vi "Controle_Manip_Main_GUI_Backup2.vi"() -> ()   [LabVIEW 2019] (continued)
                                }
                                frame #2 {
                                n2013 = local read "BackgroundSpec"() -> (w2482:dbl[])
                                n2014 = call-poly <vilib>:"Mean.vi"("X"=w2482) -> ("mean"=w2484:dbl)  [unwired: 1 out]
                                n2015 = Negate(x=w2484) -> (-x=w2483:dbl)
                                n2016 = property on="CCD 1D Spectrum Main" class="XYGraph (strict)"("YScale.Offset"=w2483) -> ()  [unwired: 2 in, 2 out]
                                }
                                frame #3 {
                                n2017 = local write "Background taken?"(TRUE ("Background taken?")) -> ()
                                n2018 = property on="Background substract" class="Enum (strict)"("Value"=enum16{"None", "Shutter"}."None" ("Background substract")) -> ()  [unwired: 2 in, 2 out]
                                }
                                }
                                }
                                frame "Image" {
                                n2019 = stacked-sequence {
                                tunnel: w2488 -> [_ w2496]
                                tunnel: w2487 -> [_ w2494]
                                frame #0 {
                                n2020 = property on="CCD 1D Spectrum Main" class="XYGraph (strict)"("Visible"=FALSE) -> ()  [unwired: 2 in, 2 out]
                                n2021 = property on="CCD 2D Image Main" class="IntGraph (strict)"("Visible"=TRUE) -> ()  [unwired: 2 in, 2 out]
                                }
                                frame #1 {
                                n2022 = local read "Wavelength calibration"() -> (w2495:dbl[])
                                n2023 = local read "CCD ROI"() -> (w2491:T20)
                                n2024 = call "PrepareData4Graph.vi"("Wavelength nm"=w2495, "DataLF"=w2496, "CCD ROI"=w2491, "AcqMode"=w2494, "Data type"=T30."Spectre") -> ("Intensity Graph"=w2493:dbl[][])  [unwired: 2 in, 3 out]
                                n2025 = local write "CCD 2D Image Main"(w2493) -> ()
                                }
                                }
                                }
                                }
                              }
                              frame True {
                              }
                            }
                          }
                          frame #1 {
                            w2521 = 1 ("Active X Scale")
                            w2522 = 0
                            # "prep axes for graphs (a nightmare in LabVIEW to not display 1...N but rather Volts or um)"
                            n2026 = local read "Scan X Res. (V)"() -> (w2526:dbl)
                            n2027 = local read "Scan X Tot. Length (V)"() -> (w2524:dbl)
                            n2028 = local read "Scan X Res. (V)"() -> (w2555:dbl)
                            n2029 = local read "Scan X Center (V)"() -> (w2523:dbl)
                            n2030 = local read "Scan X Center (V)"() -> (w2557:dbl)
                            n2031 = local read "Scan Y Center (V)"() -> (w2549:dbl)
                            n2032 = local read "Scan Y Res. (V)"() -> (w2548:dbl)
                            n2033 = local read "Scan Y Tot. Length"() -> (w2551:dbl)
                            n2034 = local read "Scan X Tot. Length (V)"() -> (w2556:dbl)
                            n2035 = local read "V2um"() -> (w2525:dbl)
                            n2036 = call "V2um.vi"("Numeric"=w2526, "V2um"=w2525) -> ("x*y"=w2530:dbl)
                            n2037 = call "V2um.vi"("Numeric"=w2524, "V2um"=w2525) -> ("x*y"=w2527:dbl)
                            n2038 = call "V2um.vi"("Numeric"=w2523, "V2um"=w2525) -> ("x*y"=w2531:dbl)
                            n2039 = Divide(x=w2527, y=w2530) -> (x/y=w2528:dbl)
                            n2040 = local read "Scan Y Res. (V)"() -> (w2537:dbl)
                            n2041 = Divide(x=w2551, y=w2548) -> (x/y=w2552:dbl)
                            n2042 = Increment(x=w2552) -> (x+1=w2550:dbl)
                            n2043 = Increment(x=w2528) -> (x+1=w2529:dbl)
                            n2044 = call "AxXYGraph.vi"("dx"=w2530, "N"=w2529, "x0"=w2531) -> ("Multiplier"=w2520:dbl, "Offset"=w2519:dbl)
                            n2045 = local read "Scan Y Tot. Length"() -> (w2539:dbl)
                            n2046 = Divide(x=w2556, y=w2555) -> (x/y=w2554:dbl)
                            n2047 = local read "Scan Y Center (V)"() -> (w2540:dbl)
                            n2048 = call "AxXYGraph.vi"("dx"=w2548, "N"=w2550, "x0"=w2549) -> ("Multiplier"=w2547:dbl, "Offset"=w2546:dbl)
                            n2049 = Increment(x=w2554) -> (x+1=w2553:dbl)
                            n2050 = call "AxXYGraph.vi"("dx"=w2555, "N"=w2553, "x0"=w2557) -> ("Multiplier"=w2544:dbl, "Offset"=w2545:dbl)
                            n2051 = local read "BackgroundSpec"() -> (w2543:dbl[])
                            n2052 = local read "V2um"() -> (w2538:dbl)
                            n2053 = call "V2um.vi"("Numeric"=w2537, "V2um"=w2538) -> ("x*y"=w2533:dbl)
                            n2054 = call "V2um.vi"("Numeric"=w2539, "V2um"=w2538) -> ("x*y"=w2536:dbl)
                            n2055 = call "V2um.vi"("Numeric"=w2540, "V2um"=w2538) -> ("x*y"=w2532:dbl)
                            n2056 = Divide(x=w2536, y=w2533) -> (x/y=w2535:dbl)
                            n2057 = Increment(x=w2535) -> (x+1=w2534:dbl)
                            n2058 = call "AxXYGraph.vi"("dx"=w2533, "N"=w2534, "x0"=w2532) -> ("Multiplier"=w2518:dbl, "Offset"=w2517:dbl)
                            n2059 = call-poly <vilib>:"Mean.vi"("X"=w2543) -> ("mean"=w2542:dbl)  [unwired: 1 out]
                            n2060 = property on="XY Intensity Map" class="IntGraph (strict)"("ActXScl"=w2522, "XScale.Multiplier"=w2544, "XScale.Offset"=w2545, "ActYScl"=w2522, "YScale.Multiplier"=w2547, "YScale.Offset"=w2546) -> ()  [unwired: 2 in, 2 out]
                            n2061 = property on="XY Intensity Map" class="IntGraph (strict)"("ActXScl"=w2521, "XScale.Multiplier"=w2520, "XScale.Offset"=w2519, "ActYScl"=w2521, "YScale.Multiplier"=w2518, "YScale.Offset"=w2517) -> ()  [unwired: 2 in, 2 out]
                            n2062 = Negate(x=w2542) -> (-x=w2541:dbl)
                            n2063 = property on="CCD 1D Spectrum XY Map" class="XYGraph (strict)"("YScale.Offset"=w2541) -> ()  [unwired: 2 in, 2 out]
                          }
                          frame #2 {
                            w2577 = 1 ("Active Y Scale")
                            w2587 = FALSE
                            w2588 = TRUE ("Visible")
                            # "nightmare part II"
                            n2064 = local read "Scan X Res. (V)"() -> (w2565:dbl)
                            n2065 = local read "Scan Y Center (V)"() -> (w2582:dbl)
                            n2066 = local read "Scan X Center (V)"() -> (w2583:dbl)
                            n2067 = local read "Scanning Mode"() -> (w2592:T21)
                            n2068 = local read "Scan Y Res. (V)"() -> (w2566:dbl)
                            n2069 = local read "Scan Fast Axis"() -> (w2593:enum16{"Y", "X"})
                            n2070 = local read "Scan XY Map Params"() -> (w2595:refnum<vi>[])
                            n2071 = property on="Save XY Map" class="Bool (strict)"("Visible"=w2587) -> ()  [unwired: 2 in, 2 out]
                            n2072 = property on="Acquire XY Map" class="Bool (strict)"("Visible"=w2587) -> ()  [unwired: 2 in, 2 out]
                            n2073 = local read "Scan X Tot. Length (V)"() -> (w2580:dbl)
                            n2074 = control-ref of="MasterPause"() -> (w2562:refnum<vi>)
                            n2075 = local read "Scan Y Tot. Length"() -> (w2581:dbl)
                            n2076 = property on="CCD 1D Spectrum Main Energy Scale" class="XYGraph (strict)"() -> ("XScale.MarkerVals[]"=w2586:dbl[], "XScale.Maximum"=w2585:dbl, "XScale.Minimum"=w2584:dbl)  [unwired: 2 in, 2 out]
                            n2077 = property on="Experiment Graph Controls" class="TabCtl (strict)"("Value"=T25."XY Intensity Map" ("Experiment Graph Controls")) -> ()  [unwired: 2 in, 2 out]
                            n2078 = property class="Bool (strict)"(reference=w2562, "Visible"=TRUE) -> ()  [unwired: 1 in, 2 out]
                            n2079 = call "Enable&Disable_Controls.vi"("Enum"=enum16{"Enabled", "Disabled", "Disabled&Grayed"}."Disabled&Grayed", "References"=w2595) -> ()  [unwired: 1 in]
                            n2080 = Bundle("Scan Fast Axis"=w2593, "Scanning Mode"=w2592, "Scan X Center (V)"=w2583, "Scan X Res. (V)"=w2565, "Scan X Tot. Length (V)"=w2580, "Scan Y Center (V)"=w2582, "Scan Y Res. (V)"=w2566, "Scan Y Tot. Length"=w2581) -> (→"Params XY Map SubVI":T23)  [unwired: 1 in]
                            n2081 = property on="Scan Main Progess Bar" class="Slide (strict)"("Visible"=TRUE, "Value"=u8 0 ("Scan XY Map Progess Bar")) -> ()  [unwired: 2 in, 2 out]
                            n2082 = control-ref of="MasterStop"() -> (w2559:refnum<vi>)
                            n2083 = local read "V2um"() -> (w2564:dbl)
                            n2084 = property on="CCD 1D XY Map Spectrum Main Energy Scale" class="XYGraph (strict)"("XScale.MarkerVals[]"=w2586, "XScale.Maximum"=w2585, "XScale.Minimum"=w2584, "XScale.UniformMarker"=TRUE ("X Scale.Uniform Marker Spacing?")) -> ()  [unwired: 2 in, 2 out]
                            n2085 = property class="Bool (strict)"(reference=w2559, "Visible"=TRUE) -> ()  [unwired: 1 in, 2 out]
                            n2086 = call "AxxXY.vi"("Y Tot"=w2581, "X Tot"=w2580, "Y Res"=w2566, "Y Center"=w2582, "X Res"=w2566, "X Center"=w2583) -> ("YMIN"=w2568:dbl, "YMAX"=w2567:dbl, "XMIN"=w2569:dbl, "XMAX"=w2570:dbl)
                            n2087 = call "V2um.vi"("Numeric"=w2569, "V2um"=w2564) -> ("x*y"=w2575:dbl)
                            n2088 = call "V2um.vi"("Numeric"=w2570, "V2um"=w2564) -> ("x*y"=w2576:dbl)
                            n2089 = call "V2um.vi"("Numeric"=w2568, "V2um"=w2564) -> ("x*y"=w2574:dbl)
                            n2090 = call "V2um.vi"("Numeric"=w2567, "V2um"=w2564) -> ("x*y"=w2573:dbl)
                            n2091 = call "V2um.vi"("Numeric"=w2566, "V2um"=w2564) -> ("x*y"=w2572:dbl)
                            n2092 = call "V2um.vi"("Numeric"=w2565, "V2um"=w2564) -> ("x*y"=w2571:dbl)
                            n2093 = property on="Elapsed (s)" class="DigNum (strict)"("Visible"=w2588) -> ()  [unwired: 2 in, 2 out]
                            n2094 = property on="Expected (s)" class="DigNum (strict)"("Visible"=w2588) -> ()  [unwired: 2 in, 2 out]
                            n2095 = property on="XY Intensity Map" class="IntGraph (strict)"("ActYScl"=0 ("Active Y Scale"), "ActXScl"=0 ("Active X Scale"), "XScale.Maximum"=w2570, "XScale.Minimum"=w2569, "YScale.Minimum"=w2568, "YScale.Maximum"=w2567, "YScale.Increment"=w2566, "XScale.Increment"=w2565) -> ()  [unwired: 2 in, 2 out]
                            n2096 = property on="XY Intensity Map" class="IntGraph (strict)"("ActYScl"=w2577, "ActXScl"=w2577, "XScale.Maximum"=w2576, "XScale.Minimum"=w2575, "YScale.Minimum"=w2574, "YScale.Maximum"=w2573, "YScale.Increment"=w2572, "XScale.Increment"=w2571) -> ()  [unwired: 2 in, 2 out]
                          }
                          frame #3 {
                            w2596 = 0 ("Active X Scale")
                            n2097 = property on="XY Intensity Map" class="IntGraph (strict)"("ActXScl"=w2596, "ActYScl"=w2596) -> ()  [unwired: 2 in, 2 out]
                          }
                          frame #4 {
                            n2098 = local read "Excitation Wavelength (nm)"() -> (w2606:dbl)
                            n2099 = local read "FSM Y Task"() -> (w2617:refnum<k21>)
                            n2100 = local read "FSM X Task"() -> (w2618:refnum<k21>)
                            n2101 = local read "Photodiode handle out"() -> (w2607:refnum<visa-resource-name>)
                            n2102 = local read "LightField Automation out"() -> (w2609:refnum<class "LightField Automation.lvclass">)
                            n2103 = local read "Photodiode error out"() -> (w2605:errorcluster)
                            n2104 = local read "Excitation Wavelength (nm)"() -> (w2613:dbl)
                            n2105 = local read "LightField Automation error out"() -> (w2608:errorcluster)
                            n2106 = local read "KCube Shutter On?"() -> (w2610:bool)
                            n2107 = local read "BackgroundSpec"() -> (w2599:dbl[])
                            n2108 = local read "Accumulations"() -> (w2614:dbl)
                            n2109 = local read "Acq Time (ms)"() -> (w2615:dbl)
                            n2110 = local read "Acq Mode"() -> (w2612:T3)
                            n2111 = local read "CCD ROI"() -> (w2611:T20)
                            n2112 = Bundle("LightField Automation out"=w2609, "LightField Automation error out"=w2608, "FSM X Task"=w2618, "FSM Y Task"=w2617) -> (→"Scan XY Map Handles":T12)  [unwired: 1 in]
                            n2113 = call <instrlib>:"TLPM Set Wavelength.vi"("error in (no error)"=w2605, "Wavelength (0.0)"=w2606, "instrument handle"=w2607) -> ("error out"=w2604:errorcluster, "instrument handle out"=w2603:refnum<visa-resource-name>)  [unwired: 7 in]
                            n2114 = call <instrlib>:"TLPM Measure Power.vi"("error in (no error)"=w2604, "instrument handle"=w2603) -> ("error out"=w2601:errorcluster, "Power"=w2600:dbl, "instrument handle out"=w2602:refnum<visa-resource-name>)  [unwired: 7 in]
                            n2115 = local write "Photodiode handle out"(w2602) -> ()
                            n2116 = local write "Photodiode error out"(w2601) -> ()
                            n2117 = local write "Excitation Power (uW)"(w2600) -> ()
                            n2118 = control-ref of="Display Mode"() -> (w2598:refnum<vi>)
                            n2119 = Bundle("Acq Time (ms)"=w2615, "Accumulations"=w2614, "Excitation Wavelength (nm)"=w2613, "Acq Mode"=w2612, "CCD ROI"=w2611, "KCube Shutter On?"=w2610, "Power"=w2600, "BackgroundSpec"=w2599, "Display Mode"=w2598) -> (→"Scan XY Map Exp Params SubVI":T7)  [unwired: 1 in]
                            n2120 = case shown="True" w2610 {
                              selector: w2610 -> [_ w2619]
                              frame False {
                              }
                              frame True {
                                n2121 = control-ref of="Shutter Ctrls"() -> (w2622:refnum<vi>)
                                n2122 = property class="Ring (strict)"(reference=w2622) -> ("Value"=w2623:u16)  [unwired: 1 in, 2 out]
                                n2123 = control-ref of="KCube Shutter Device Reference"() -> (w2621:refnum<vi>)
                                n2124 = Equal?(x=w2623, y=u16 0) -> (x = y?=w2624:bool)
                                n2125 = case shown="True" w2624 {
                                tunnel: w2621 -> [_ w2627]
                                tunnel: w2622 -> [_ w2626]
                                tunnel: w2619 -> [_ w2625]
                                frame False {
                                }
                                frame True {
                                n2126 = call "Shutter.vi"("KCube Shutter Device Reference 2"=w2627, "Shutter Ctrls 2"=w2626, "Shutter on?"=w2625) -> ()
                                }
                                }
                              }
                            }
                          }
                          frame #5 {
                            n2127 = local read "Scan XY Map Exp Params SubVI"() -> (w2630:T7)
                            n2128 = local read "Scan XY Map References"() -> (w2631:T9)
                            n2129 = local read "Params XY Map SubVI"() -> (w2635:T23)
                            n2130 = local read "Scan XY Map Handles"() -> (w2634:T12)
                            n2131 = call "ScanFSM_v2.vi"("Scan XY Map References"=w2631, "Scan XY Map Handles"=w2634, "Params XY Map SubVI"=w2635, "Scan XY Map Exp Params SubVI"=w2630) -> ("Handles Out"=w2632:T36, "Data"=w2633:i32[][], "XYPos Indices"=w2629:i32[][], "XYPositions"=→"XYPositions":dbl[][])  [unwired: 12 in]
                            n2132 = local write "Scan XY Map Handles"(w2632) -> ()
                            n2133 = local write "XYMap Data"(w2633) -> ()
                            n2134 = local write "XYPos Indices"(w2629) -> ()
                          }
                          frame #6 {
                            n2135 = local read "Scan XY Map Handles"() -> (w2641:T12)
                            n2136 = local read "Scan Y Center (V)"() -> (w2636:dbl)
                            n2137 = local read "Scan X Center (V)"() -> (w2638:dbl)
                            n2138 = local read "KCube Shutter On?"() -> (w2643:bool)
                            n2139 = control-ref of="Shutter Ctrls"() -> (w2645:refnum<vi>)
                            n2140 = local read "FSM X Task"() -> (w2642:refnum<k21>)
                            n2141 = local read "FSM Y Task"() -> (w2637:refnum<k21>)
                            n2142 = control-ref of="KCube Shutter Device Reference"() -> (w2644:refnum<vi>)
                            n2143 = call "Shutter.vi"("KCube Shutter Device Reference 2"=w2644, "Shutter Ctrls 2"=w2645, "Shutter on?"=w2643) -> ()
                            n2144 = call "FSMGoTo.vi"("Target Value (V)"=w2638, "FSM Task"=w2642) -> ()  [unwired: 1 out]
                            n2145 = call "FSMGoTo.vi"("Target Value (V)"=w2636, "FSM Task"=w2637) -> ()  [unwired: 1 out]
                            n2146 = local write "Scan X Readout (V)"(w2638) -> ()
                            n2147 = Unbundle By Name(w2641) -> ("LightField Automation out"=w2640:refnum<class "LightField Automation.lvclass">, "LightField Automation error out"=w2639:errorcluster)
                            n2148 = property on="XY Intensity Map" class="IntGraph (strict)"("Cursor.Cursor X"=w2638) -> ()  [unwired: 2 in, 2 out]
                            n2149 = local write "Scan Y Readout (V)"(w2636) -> ()
                            n2150 = property on="XY Intensity Map" class="IntGraph (strict)"("Cursor.Cursor Y"=w2636) -> ()  [unwired: 2 in, 2 out]
                            n2151 = local write "LightField Automation error out"(w2639) -> ()
                            n2152 = local write "LightField Automation out"(w2640) -> ()
                          }
                          frame #7 {
                            w2646 = T28."Disabled and Grayed Out" ("Disabled")
                            w2659 = FALSE ("Visible")
                            n2153 = local read "Scan XY Map Params"() -> (w2663:refnum<vi>[])
                            n2154 = local read "Auto< ?"() -> (w2652:bool)
                            n2155 = local write "Acquire XY Map"(FALSE ("Acquire XY Map")) -> ()
                            n2156 = local write "Save XY Map"(FALSE ("Acquire XY Map")) -> ()
                            n2157 = case shown="True" w2652 {
                              tunnel: [TRUE FALSE] -> w2651
                              frame False {
                              }
                              frame True {
                              }
                            }
                            n2158 = call "Enable&Disable_Controls.vi"("Enum"=enum16{"Enabled", "Disabled", "Disabled&Grayed"}."Enabled", "References"=w2663) -> ()  [unwired: 1 in]
                            n2159 = property on="Acquire XY Map" class="Bool (strict)"("Visible"=TRUE, "Value"=FALSE ("Acquire XY Map")) -> ()  [unwired: 2 in, 2 out]
                            n2160 = local write "ExportMapPosition?"(TRUE ("ExportMapPosition?")) -> ()
                            n2161 = disable-structure shown="Disabled" {
                              disable-tunnel: w2659 -> [w2666 _]
                              frame Disabled {
                                n2162 = property on="Scan Main Progess Bar" class="Slide (strict)"("Visible"=w2666) -> ()  [unwired: 2 in, 2 out]
                              }
                              frame Enabled {
                              }
                            }
                            n2163 = property on="Save XY Map" class="Bool (strict)"("Visible"=w2651) -> ()  [unwired: 2 in, 2 out]
                            n2164 = property on="Elapsed (s)" class="DigNum (strict)"("Visible"=w2659) -> ("Value"=w2649:dbl)  [unwired: 2 in, 2 out]
                            n2165 = control-ref of="MasterStop"() -> (w2654:refnum<vi>)
                            n2166 = control-ref of="Scanning Mode"() -> (w2648:refnum<vi>)
                            n2167 = control-ref of="Scan Fast Axis"() -> (w2647:refnum<vi>)
                            n2168 = control-ref of="MasterPause"() -> (w2655:refnum<vi>)
                            n2169 = local write "Scan Main Progess Bar"(u8 0 ("Scan Main Progess Bar")) -> ()
                            n2170 = control-ref of="ExperimentStopped?"() -> (w2653:refnum<vi>)
                            n2171 = call "CheckStopAndReset.vi"("ExperimentStopped?"=w2653, "MasterStop"=w2654, "MasterPause"=w2655) -> ()
                            n2172 = property on="Expected (s)" class="DigNum (strict)"("Value"=w2649) -> ()  [unwired: 2 in, 2 out]
                            n2173 = property class="Enum (strict)"(reference=w2647, "DisabledEnum"=w2646) -> ()  [unwired: 1 in, 2 out]
                            n2174 = property class="Enum (strict)"(reference=w2648, "DisabledEnum"=w2646) -> ()  [unwired: 1 in, 2 out]
                          }
                        }
                      }
                      frame "Acquire Contrast test array of references" {
                        n2175 = stacked-sequence {
                          frame #0 {
                            w2669 = FALSE
                            w2670 = TRUE
                            w2678 = FALSE ("Acq Cont")
                            w2675 = FALSE ("Acq Cont")
                            n2176 = property on="CCD 1D Spectrum Main" class="XYGraph (strict)"() -> ("XScale.Maximum"=w2674:dbl, "XScale.Minimum"=w2673:dbl, "YScale.Minimum"=w2672:dbl, "YScale.Maximum"=w2671:dbl)  [unwired: 2 in, 2 out]
                            n2177 = property on="Acquire Contrast" class="Bool (strict)"("Visible"=w2669) -> ()  [unwired: 2 in, 2 out]
                            n2178 = property on="Save Contrast" class="Bool (strict)"("Visible"=w2669) -> ()  [unwired: 2 in, 2 out]
                            n2179 = property on="Scan Linear Stage Progess Bar" class="Slide (strict)"("Visible"=TRUE, "Value"=u8 0 ("Scan Linear Stage Progess Bar")) -> ()  [unwired: 2 in, 2 out]
                            n2180 = property on="Pause Contrast" class="Bool (strict)"("Visible"=w2670) -> ()  [unwired: 2 in, 2 out]
                            n2181 = property on="Stop Contrast" class="Bool (strict)"("Visible"=w2670) -> ()  [unwired: 2 in, 2 out]
                            n2182 = property on="Contrast 1D Spectrum" class="XYGraph (strict)"("XScale.Maximum"=w2674, "XScale.Minimum"=w2673, "YScale.Minimum"=w2672, "YScale.Maximum"=w2671) -> ()  [unwired: 2 in, 2 out]
                            n2183 = local read "Scan Contrast Ctrls"() -> (w2679:refnum<vi>[])
                            n2184 = property on="Experiment Graph Controls" class="TabCtl (strict)"("Value"=T25."Contrast" ("Experiment Graph Controls")) -> ()  [unwired: 2 in, 2 out]
                            n2185 = property on="Scan Linear Stage Progess Bar" class="Slide (strict)"("Visible"=TRUE) -> ()  [unwired: 2 in, 2 out]
                            n2186 = call "Enable&Disable_Controls.vi"("Enum"=enum16{"Enabled", "Disabled", "Disabled&Grayed"}."Disabled&Grayed", "References"=w2679) -> ()  [unwired: 1 in]
                            n2187 = local write "Acquire Contrast"(w2675) -> ()
                            n2188 = local write "Save Contrast"(w2675) -> ()
                            n2189 = local write "Pause Contrast"(w2678) -> ()
                            n2190 = local write "Stop Contrast"(w2678) -> ()
                          }
                          frame #1 {
                            n2191 = local read "ESP 301 COM Port"() -> (w2694:refnum<visa-resource-name>)
                            n2192 = local read "Photodiode handle out"() -> (w2692:refnum<visa-resource-name>)
                            n2193 = local read "Photodiode error out"() -> (w2691:errorcluster)
                            n2194 = local read "LightField Automation error out"() -> (w2681:errorcluster)
                            n2195 = local read "LinTFine End Pos (usteps)"() -> (w2698:dbl)
                            n2196 = local read "LinTFines Step Pos (usteps)"() -> (w2699:dbl)
                            n2197 = local read "LinTFine Start Pos (usteps)"() -> (w2700:dbl)
                            n2198 = local read "PZC200 Instrument Channel"() -> (w2696:string)
                            n2199 = local read "LinT End pos (mm)"() -> (w2701:dbl)
                            n2200 = local read "LightField Automation out"() -> (w2682:refnum<class "LightField Automation.lvclass">)
                            n2201 = local read "LinT Step Pos (mm)"() -> (w2702:dbl)
                            n2202 = local read "LinT Start Pos (mm)"() -> (w2703:dbl)
                            n2203 = local read "ESP 301 Error"() -> (w2693:errorcluster)
                            n2204 = local read "PZC Error"() -> (w2695:errorcluster)
                            n2205 = Bundle("LinT Start Pos (mm)"=w2703, "LinT Step Pos (mm)"=w2702, "LinT End pos (mm)"=w2701, "LinTFine Start Pos (usteps)"=w2700, "LinTFines Step Pos (usteps)"=w2699, "LinTFine End Pos (usteps)"=w2698) -> (w2697:T27)  [unwired: 1 in]
                            n2206 = local read "Excitation Wavelength (nm)"() -> (w2687:dbl)
                            n2207 = Bundle("LightField Automation out"=w2682, "LightField Automation error out"=w2681, "PZC200 Instrument Channel"=w2696, "PZC Error"=w2695, "ESP 301 COM Port"=w2694, "ESP 301 Error"=w2693, "Photodiode handle out"=w2692, "Photodiode error out"=w2691) -> (w2690:T13)  [unwired: 1 in]
                            n2208 = local read "Exposure Time (ms)"() -> (w2689:dbl)
                            n2209 = local read "KCube Shutter On?"() -> (w2683:bool)
                            n2210 = local read "Accumulations"() -> (w2688:dbl)
                            n2211 = local read "Acq Mode"() -> (w2686:T3)
                            n2212 = local read "CCD ROI"() -> (w2685:T20)
                            n2213 = local write "Scan Translation Params"(w2697) -> ()
                            n2214 = local write "Constrast Handles"(w2690) -> ()
                            n2215 = Bundle("Exposure Time (ms)"=w2689, "Accumulations"=w2688, "Excitation Wavelength (nm)"=w2687, "Acq Mode"=w2686, "CCD ROI"=w2685, "KCube Shutter On?"=w2683) -> (w2684:T24)  [unwired: 1 in]
                            n2216 = local write "Scan Translation Exp Params"(w2684) -> ()
                          }
                          frame #2 {
                            n2217 = local read "Scan Translation Exp Params"() -> (w2708:T24)
                            n2218 = local read "Contrast References"() -> (w2707:T14)
                            n2219 = local read "Scan Translation Params"() -> (w2709:T27)
                            n2220 = local read "Constrast Handles"() -> (w2710:T13)
                            n2221 = call "FineContrast_v3.0.vi"("Contrast References"=w2707, "Constrast Handles"=w2710, "Scan Translation Exp Params"=w2708, "Scan Translation Params"=w2709) -> ("Constrast Handles Out"=w2706:T37)  [unwired: 2 out]
                            n2222 = Unbundle By Name(w2706) -> ("LightField Automation out"=w2705:refnum<class "LightField Automation.lvclass">, "error out"=w2704:errorcluster)
                            n2223 = local write "Constrast Handles"(w2706) -> ()
                            n2224 = local write "LightField Automation error out"(w2704) -> ()
                            n2225 = local write "LightField Automation out"(w2705) -> ()
                          }
                          frame #3 {
                            w2712 = TRUE
                            w2711 = FALSE
                            w2716 = FALSE ("Acq Cont")
                            w2713 = FALSE ("Acq Cont")
                            n2226 = property on="Scan Linear Stage Progess Bar" class="Slide (strict)"("Visible"=FALSE, "Value"=u8 0 ("Scan Linear Stage Progess Bar")) -> ()  [unwired: 2 in, 2 out]
                            n2227 = property on="Acquire Contrast" class="Bool (strict)"("Visible"=w2712) -> ()  [unwired: 2 in, 2 out]
                            n2228 = property on="Save Contrast" class="Bool (strict)"("Visible"=w2712) -> ()  [unwired: 2 in, 2 out]
                            n2229 = property on="Pause Contrast" class="Bool (strict)"("Visible"=w2711) -> ()  [unwired: 2 in, 2 out]
                            n2230 = property on="Stop Contrast" class="Bool (strict)"("Visible"=w2711) -> ()  [unwired: 2 in, 2 out]
                            n2231 = local read "Scan Contrast Ctrls"() -> (w2717:refnum<vi>[])
                            n2232 = local write "Acquire Michelson"(w2713) -> ()
                            n2233 = local write "Acquire Contrast"(w2713) -> ()
                            n2234 = local write "Save Michelson"(w2713) -> ()
                            n2235 = local write "Pause Michelson"(w2716) -> ()
                            n2236 = local write "Stop Michelson"(w2716) -> ()
                            n2237 = call "Enable&Disable_Controls.vi"("Enum"=enum16{"Enabled", "Disabled", "Disabled&Grayed"}."Enabled", "References"=w2717) -> ()  [unwired: 1 in]
                          }
                        }
                      }
                      frame "Acquire Contrast EVERYTHING OK" {
                        n2238 = stacked-sequence {
                          tunnel: [_ w2734 _] -> _
                          frame #0 {
                            w2726 = FALSE
                            w2729 = TRUE
                            n2239 = property on="Stop Contrast" class="Bool (strict)"("Visible"=w2729) -> ()  [unwired: 2 in, 2 out]
                            n2240 = property on="Pause Contrast" class="Bool (strict)"("Visible"=w2729) -> ()  [unwired: 2 in, 2 out]
                            n2241 = property on="Experiment Graph Controls" class="TabCtl (strict)"("Value"=T25."Contrast" ("Experiment Graph Controls")) -> ()  [unwired: 2 in, 2 out]
                            n2242 = local read "Scan Contrast Ctrls"() -> (w2727:refnum<vi>[])
                            n2243 = property on="Save Contrast" class="Bool (strict)"("Visible"=w2726) -> ()  [unwired: 2 in, 2 out]
                            n2244 = property on="Acquire Contrast" class="Bool (strict)"("Visible"=w2726) -> ()  [unwired: 2 in, 2 out]
                            n2245 = call "Enable&Disable_Controls.vi"("Enum"=enum16{"Enabled", "Disabled", "Disabled&Grayed"}."Disabled&Grayed", "References"=w2727) -> ()  [unwired: 1 in]
                            n2246 = property on="CCD 1D Spectrum Main" class="XYGraph (strict)"() -> ("XScale.Maximum"=w2725:dbl, "XScale.Minimum"=w2724:dbl, "YScale.Minimum"=w2723:dbl, "YScale.Maximum"=w2722:dbl)  [unwired: 2 in, 2 out]
                            n2247 = property on="Scan Linear Stage Progess Bar" class="Slide (strict)"("Visible"=TRUE, "Value"=u8 0 ("Scan Linear Stage Progess Bar")) -> ()  [unwired: 2 in, 2 out]
                            n2248 = property on="Contrast 1D Spectrum" class="XYGraph (strict)"("XScale.Maximum"=w2725, "XScale.Minimum"=w2724, "YScale.Minimum"=w2723, "YScale.Maximum"=w2722) -> ()  [unwired: 2 in, 2 out]
                          }
                          frame #1 {
                            n2249 = local read "Excitation Wavelength (nm)"() -> (w2738:dbl)
                            n2250 = local read "LinTFines Step Pos (usteps)"() -> (w2742:dbl)
                            n2251 = local read "LinTFine Start Pos (usteps)"() -> (w2744:dbl)
                            n2252 = local read "LinTFine End Pos (usteps)"() -> (w2743:dbl)
                            n2253 = local read "Exposure Time (ms)"() -> (w2740:dbl)
                            n2254 = local read "LightField Automation error out"() -> (w2730:errorcluster)
                            n2255 = local read "Acq Mode"() -> (w2739:T3)
                            n2256 = local read "CCD ROI"() -> (w2734:T20)
                            n2257 = local read "LightField Automation out"() -> (w2731:refnum<class "LightField Automation.lvclass">)
                            n2258 = control-ref of="KCube Shutter Device Reference"() -> (w2746:refnum<vi>)
                            n2259 = control-ref of="PZC Position Readout (usteps)"() -> (w2753:refnum<vi>)
                            n2260 = control-ref of="Scan Linear Stage Progess Bar"() -> (w2752:refnum<vi>)
                            n2261 = local read "PZC200 Instrument Channel"() -> (w2745:string)
                            n2262 = control-ref of="Contrast Oscillations"() -> (w2750:refnum<vi>)
                            n2263 = control-ref of="Pause Contrast"() -> (w2751:refnum<vi>)
                            n2264 = control-ref of="Contrast 1D Spectrum"() -> (w2749:refnum<vi>)
                            n2265 = Open VI Reference(type specifier VI Refnum (for type only)=refnum<vi> refnum ("application reference (local)"), vi path=path "D:/Users/manip-thz/Documents/Controle_Manip_2020/subVIs/Scans/FineContrast.vi", options=256) -> (vi reference=w2760:refnum<vi>, error out=w2759:errorcluster)  [unwired: 3 in]
                            n2266 = control-ref of="Stop Contrast"() -> (w2748:refnum<vi>)
                            n2267 = local read "PZC Error"() -> (w2754:errorcluster)
                            n2268 = control-ref of="Shutter Ctrls"() -> (w2747:refnum<vi>)
                            n2269 = call-by-ref "Wait On Asynchronous Call"(reference=w2760, error in=w2759) -> (reference out=w2756:refnum<vi>, error out=w2755:errorcluster, "LightField Automation out"=w2732:refnum<class "LightField Automation.lvclass">, "PZC200 Instrument Channel 2"=w2758:string, "PZC Error 2"=w2757:errorcluster, "PZAPos & InstPow"=w2735:dbl[][], "Spectra vs PZA"=w2741:i32[][], "LightField Automation error  out"=w2733:errorcluster)  [unwired: 22 in]
                            n2270 = local write "PZAPos&Pow"(w2735) -> ()
                            n2271 = Close Reference(reference=w2756, error in (no error)=w2755) -> ()  [unwired: 1 out]
                            n2272 = local write "PZC Error"(w2757) -> ()
                            n2273 = local write "Contrast Array Out"(w2741) -> ()
                            n2274 = local write "PZC200 Instrument Channel"(w2758) -> ()
                            n2275 = local read "Photodiode handle out"() -> (w2736:refnum<visa-resource-name>)
                            n2276 = local read "Photodiode error out"() -> (w2737:errorcluster)
                            n2277 = call-by-ref "Start Asynchronous Call"(reference=w2760, error in=w2759, "LightField Automation"=w2731, "PZC200 Instrument Channel"=w2745, "ExcWL_nm"=w2738, "PZC Error"=w2754, "Acq Time (ms) 2"=w2740, "Acq Mode"=w2739, "CCD ROI"=w2734, "LightField Automation error"=w2730, "Shutter Device Reference"=w2746, "PZC Position Readout (usteps) 2"=w2753, "LinTFine Start"=w2744, "LinTFine End"=w2743, "Shutter Controls"=w2747, "Scan Spectrum Progess Bar 2"=w2752, "Stop Contrast 2"=w2748, "Pause Contrast 2"=w2751, "Contrast 1D Spectrum 2"=w2749, "LinTFine Step"=w2742, "Contrast Oscillations 2"=w2750, "Photodiode handle out"=w2736, "Photodiode error out"=w2737) -> ()  [unwired: 1 in, 8 out]
                            n2278 = local write "LightField Automation error out"(w2733) -> ()
                            n2279 = local write "LightField Automation out"(w2732) -> ()
                          }
                          frame #2 {
                            w2767 = FALSE ("Acq Cont")
                            w2764 = FALSE ("Acq Cont")
                            w2768 = TRUE
                            w2771 = FALSE
                            n2280 = property on="Stop Contrast" class="Bool (strict)"("Visible"=w2771) -> ()  [unwired: 2 in, 2 out]
                            n2281 = property on="Pause Contrast" class="Bool (strict)"("Visible"=w2771) -> ()  [unwired: 2 in, 2 out]
                            n2282 = local read "Scan Contrast Ctrls"() -> (w2769:refnum<vi>[])
                            n2283 = property on="Save Contrast" class="Bool (strict)"("Visible"=w2768) -> ()  [unwired: 2 in, 2 out]
                            n2284 = property on="Acquire Contrast" class="Bool (strict)"("Visible"=w2768) -> ()  [unwired: 2 in, 2 out]
                            n2285 = call "Enable&Disable_Controls.vi"("Enum"=enum16{"Enabled", "Disabled", "Disabled&Grayed"}."Enabled", "References"=w2769) -> ()  [unwired: 1 in]
                            n2286 = local write "Acquire Contrast"(w2764) -> ()
                            n2287 = local write "Save Contrast"(w2764) -> ()
                            n2288 = local write "Pause Contrast"(w2767) -> ()
                            n2289 = local write "Stop Contrast"(w2767) -> ()
                            n2290 = property on="Scan Linear Stage Progess Bar" class="Slide (strict)"("Visible"=TRUE, "Value"=u8 0 ("Scan Linear Stage Progess Bar")) -> ()  [unwired: 2 in, 2 out]
                          }
                        }
                      }
                    }
                  }
                }
              }
              frame #1 {
                # "AutoSave?"
                n2291 = local read "ExperimentStopped?"() -> (w2774:bool)
                n2292 = property class="Bool"(reference=w2777) -> ("Label.Text"=w2776:string)  [unwired: 1 in, 2 out]
                n2293 = Not(x=w2774) -> (.not. x?=w2773:bool)
                n2294 = local read "Auto< ?"() -> (w2775:bool)
                n2295 = And(x=w2775, y=w2773) -> (x .and. y?=w2772:bool)
                "x .and. y?" <- w2772
                n2296 = case shown="True" w2772 {
                  tunnel: w2776 -> [_ w2778]
                  frame False {
                  }
                  frame True {
                    n2297 = case shown="\"Acquire PLE\"" w2778 {
                      frame "Acquire Continuous Spectrum" {
                      }
                      frame "Fast Acq Continuous" {
                      }
                      frame "Acquire Polarisation" {
                        n2298 = property on="Save Polarisation" class="Bool (strict)"("Val(Sgnl)"=TRUE ("Value (Signaling)")) -> ()  [unwired: 2 in, 2 out]
                      }
                      frame "Acquire fPow" {
                        n2299 = property on="Save fPow" class="Bool (strict)"("Val(Sgnl)"=TRUE ("Value (Signaling)")) -> ()  [unwired: 2 in, 2 out]
                      }
                      frame "Acquire XY Map" {
                        n2300 = property on="Save XY Map" class="Bool (strict)"("Val(Sgnl)"=TRUE ("Value (Signaling)")) -> ()  [unwired: 2 in, 2 out]
                      }
                      frame "Acquire Contrast" {
                        n2301 = property on="Save Contrast" class="Bool (strict)"("Val(Sgnl)"=TRUE ("Value (Signaling)")) -> ()  [unwired: 2 in, 2 out]
                      }
                      frame "Acquire Time Trace" {
                        n2302 = property on="Save Spectrum N" class="Bool (strict)"("Val(Sgnl)"=TRUE ("Value (Signaling)")) -> ()  [unwired: 2 in, 2 out]
                      }
                      frame Default {
                      }
                      frame "Acquire Custom Diode Spectrum" {
                        n2303 = property on="Save Custom Diode Spectrum" class="Bool (strict)"("Val(Sgnl)"=TRUE) -> ()  [unwired: 2 in, 2 out]
                      }
                      frame "Acquire PLE" {
                        n2304 = property on="Save PLE" class="Bool (strict)"("Val(Sgnl)"=TRUE ("Value (Signaling)")) -> ()  [unwired: 2 in, 2 out]
                      }
                      frame "Acquire Michelson" {
                        n2305 = property on="Save Michelson" class="Bool (strict)"("Val(Sgnl)"=TRUE ("Value (Signaling)")) -> ()  [unwired: 2 in, 2 out]
                      }
                      frame "Acquire Spectrum" {
                        n2306 = property on="Save Spectrum" class="Bool (strict)"("Val(Sgnl)"=TRUE ("Value (Signaling)")) -> ()  [unwired: 2 in, 2 out]
                      }
                      frame "Fast Acq" {
                      }
                    }
                  }
                }
              }
            }
          }
          event "Doc Cryostat", "Doc LLTF", "Doc ESP 301", "Doc Shutter", "Doc PZC200", "Doc NanoMax", "Doc Attocubes", "Doc LightField", "Doc PicoHarp", "Doc Photodiode", "Doc ESP 300", "Doc FSM": Mouse Down {
            n2307 = event-data() -> ("CtlRef"=w2793:refnum<vi>)  [unwired: 1 in, 7 out]
            n2308 = property class="Bool (strict)"(reference=w2793) -> ("Label.Text"=w2792:string)  [unwired: 1 in, 2 out]
            n2309 = case shown="\"Doc LightField\"" w2792 {
              tunnel: ["\"C:\\Users\\manip\\Documents\\Controle_Manip_2020\\Documentation\\Attocubes\\Positioners\\Manual_FlexPositioners_&_Scanner_v2.2.pdf\"" "\"C:\\Users\\manip\\Documents\\Controle_Manip_2020\\subVIs\\Light Field\\LightField-Users-Manual-Issue-4.5-4411-0125.pdf\"" "\"C:\\Users\\manip\\Documents\\Controle_Manip_2020\\subVIs\\Newport\\NanoPZ-User-Manual-RevA.pdf\"" "\"C:\\Users\\manip\\Documents\\Controle_Manip_2020\\subVIs\\Kinesis\\MAX312D_M-Manual.pdf\"" "\"C:\\Users\\manip\\Documents\\Controle_Manip_2020\\subVIs\\PicoHarp\\Manual.pdf\" " ("command line") "\"C:\\Users\\manip\\Documents\\Controle_Manip_2020\\subVIs\\TLPM\\PM16-121-SpecSheet.pdf\"" "\"C:\\Cryostation\\Help.pdf\"" "\"C:\\Users\\manip\\Desktop\\Photon etc\\PHySpec\\manuals\\LLTF Getting started 1.14.pdf\"" "\"C:\\Newport\\Motion Control\\ESP301\\Doc\\ESP301 - Controller GUI Manual.pdf\"" "\"C:\\Users\\manip\\Documents\\Controle_Manip_2020\\subVIs\\Newport\\Newport ESP300\\ESP300.pdf\"" "\"C:\\Users\\manip\\Documents\\Controle_Manip_2020\\subVIs\\Kinesis\\SH05_M-Manual.pdf\"" "\"C:\\Users\\manip\\Documents\\Controle_Manip_2020\\Documentation\\Misc\\FSM-300UserManual.pdf\""] -> w2788
              frame "Doc Attocubes" {
              }
              frame "Doc LightField" {
              }
              frame "Doc PZC200" {
              }
              frame "Doc NanoMax" {
              }
              frame "Doc PicoHarp" {
              }
              frame "Doc Photodiode" {
              }
              frame "Doc Cryostat", Default {
              }
              frame "Doc LLTF" {
              }
              frame "Doc ESP 301" {
              }
              frame "Doc ESP 300" {
              }
              frame "Doc Shutter" {
              }
              frame "Doc FSM" {
              }
            }
            n2310 = Concatenate Strings("\"C:\\Program Files\\Adobe\\Acrobat DC\\Acrobat\\Acrobat.exe\" " ("command line"), w2788) -> (w2790:string)
            n2311 = call <vilib>:"System Exec.vi"("wait until completion? (T)"=FALSE, "command line"=w2790) -> ()  [unwired: 6 in, 4 out]
          }
          event "PLE Start (nm)", "PLE End (nm)", "PLE Step (nm)": Value Change {
            n2312 = event-data() -> ()  [unwired: 1 in, 6 out]
            n2313 = local read "PLE End (nm)"() -> (w2812:dbl)
            n2314 = local read "PLE Step (nm)"() -> (w2809:dbl)
            n2315 = local read "PLE Start (nm)"() -> (w2811:dbl)
            n2316 = Subtract(x=w2812, y=w2811) -> (x-y=w2810:dbl)
            n2317 = local read "Acq Time (ms)"() -> (w2816:dbl)
            n2318 = Divide(x=w2810, y=w2809) -> (x/y=w2817:dbl)
            n2319 = Add(x=w2816, y=200.0) -> (x+y=w2815:dbl)
            n2320 = Increment(x=w2817) -> (x+1=w2808:dbl)
            "PLE # Pts" <- w2808
            n2321 = Divide(x=w2815, y=1000.0) -> (x/y=w2807:dbl)
            n2322 = Multiply(x=w2808, y=w2807) -> (x*y=w2806:dbl)
            n2323 = control-ref of="Expected (s)"() -> (w2818:refnum<vi>)
            n2324 = property class="DigNum (strict)"(reference=w2818, "Value"=w2806) -> ()  [unwired: 1 in, 2 out]
          }
          event "Display Mode": Value Change {
            n2325 = event-data() -> ("CtlRef"=w2820:refnum<vi>)  [unwired: 1 in, 5 out]
            n2326 = property class="Ring (strict)"(reference=w2820) -> ("Label.Text"=w2819:string)  [unwired: 1 in, 2 out]
            n2327 = case shown="\"Display Mode\"" w2819 {
              frame "False", Default {
              }
              frame "Display Mode" {
                n2328 = local read "Excitation Power (uW)"() -> (w2823:dbl)
                n2329 = local read "BackgroundSpec"() -> (w2824:dbl[])
                n2330 = local read "Acq Time (ms)"() -> (w2822:dbl)
                n2331 = property on="CCD 1D Spectrum Main" class="XYGraph (strict)"() -> ("Value"=w2826:cluster{dbl[], dbl[]})  [unwired: 2 in, 2 out]
                n2332 = local read "Display Mode"() -> (w2827:u16)
                n2333 = Unbundle(w2826) -> (w2825:dbl[])  [unwired: 1 out]
                n2334 = control-ref of="Cnts"() -> (w2821:refnum<vi>)
                n2335 = call "2Cnts.vi"("Array Background"=w2824, "Pow W"=w2823, "AcqTime ms"=w2822, "Cnts Ref"=w2821, "Display Mode"=w2827, "Array"=w2825) -> ()  [unwired: 1 out]
              }
            }
          }
          event "Spectrum Custom Mode": Value Change {
            # "make sure proper input before calibration"
            n2336 = event-data() -> ("NewVal"=w2832:u16)  [unwired: 1 in, 5 out]
            n2337 = case shown="2" w2832 {
              tunnel: [350.0 350.0 350.0 350.0 350.0] -> w2829
              tunnel: [900.0 900.0 900.0 900.0 900.0] -> w2828
              frame 0, Default {
              }
              frame 1 {
              }
              frame 3 {
              }
              frame 2 {
              }
              frame 4 {
              }
            }
            n2338 = control-ref of="Spectrum Start Wavelength (nm)"() -> (w2831:refnum<vi>)
            n2339 = control-ref of="Spectrum End Wavelength (nm)"() -> (w2830:refnum<vi>)
            n2340 = property class="DigNum (strict)"(reference=w2830, "Maximum"=w2828, "Minimum"=w2829) -> ()  [unwired: 1 in, 2 out]
            n2341 = property class="DigNum (strict)"(reference=w2831, "Maximum"=w2828, "Minimum"=w2829) -> ()  [unwired: 1 in, 2 out]
          }
          event Value Change {
            # "APD, CCD Image or binned CCD image"
            n2342 = event-data() -> ()  [unwired: 1 in, 6 out]
            n2343 = local read "Acq Mode"() -> (w2844:T3)
            n2344 = case shown="\"Image\"" w2844 {
              frame "Image" {
                w2846 = TRUE
                w2847 = FALSE
                n2345 = property on="CCD 1D Spectrum XY Map" class="WFGraph (strict)"("Visible"=w2847) -> ()  [unwired: 2 in, 2 out]
                n2346 = property on="CCD 1D Spectrum Main" class="XYGraph (strict)"("Visible"=w2847) -> ()  [unwired: 2 in, 2 out]
                n2347 = property on="Background substract" class="Enum (strict)"("Visible"=w2846) -> ()  [unwired: 2 in, 2 out]
                n2348 = property on="CCD ROI" class="Enum (strict)"("Visible"=w2846) -> ()  [unwired: 2 in, 2 out]
                n2349 = property on="Exit mirror" class="Ring (strict)"("Val(Sgnl)"=u16 4 ("Value (Signaling)")) -> ()  [unwired: 2 in, 2 out]
                n2350 = property on="Accumulations" class="DigNum (strict)"("Visible"=w2846) -> ()  [unwired: 2 in, 2 out]
                n2351 = property on="CCD 2D Image Main" class="IntGraph (strict)"("Visible"=w2846) -> ()  [unwired: 2 in, 2 out]
                n2352 = property on="CCD 2D Image XY Map" class="IntGraph (strict)"("Visible"=w2846) -> ()  [unwired: 2 in, 2 out]
                n2353 = property on="Exposure Time (ms)" class="DigNum (strict)"("Visible"=w2846) -> ()  [unwired: 2 in, 2 out]
              }
              frame "Spectrum" {
                w2850 = FALSE
                w2849 = TRUE
                n2354 = property on="Exit mirror" class="Ring (strict)"("Val(Sgnl)"=u16 4 ("Value (Signaling)")) -> ()  [unwired: 2 in, 2 out]
                n2355 = property on="CCD 2D Image XY Map" class="IntGraph (strict)"("Visible"=w2850) -> ()  [unwired: 2 in, 2 out]
                n2356 = property on="CCD 2D Image Main" class="IntGraph (strict)"("Visible"=w2850) -> ()  [unwired: 2 in, 2 out]
                n2357 = property on="Background substract" class="Enum (strict)"("Visible"=w2849) -> ()  [unwired: 2 in, 2 out]
                n2358 = property on="CCD ROI" class="Enum (strict)"("Visible"=w2849) -> ()  [unwired: 2 in, 2 out]
                n2359 = property on="Accumulations" class="DigNum (strict)"("Visible"=w2849) -> ()  [unwired: 2 in, 2 out]
                n2360 = property on="CCD 1D Spectrum XY Map" class="WFGraph (strict)"("Visible"=w2849) -> ()  [unwired: 2 in, 2 out]
                n2361 = property on="Exposure Time (ms)" class="DigNum (strict)"("Visible"=w2849) -> ()  [unwired: 2 in, 2 out]
                n2362 = property on="CCD 1D Spectrum Main" class="XYGraph (strict)"("Visible"=w2849) -> ()  [unwired: 2 in, 2 out]
              }
              frame "APD 1" {
                w2852 = FALSE
                w2853 = TRUE
                n2363 = property on="CCD 1D Spectrum XY Map" class="WFGraph (strict)"("Visible"=w2853) -> ()  [unwired: 2 in, 2 out]
                n2364 = property on="CCD 1D Spectrum Main" class="XYGraph (strict)"("Visible"=w2853) -> ()  [unwired: 2 in, 2 out]
                n2365 = property on="Exit mirror" class="Ring (strict)"("Val(Sgnl)"=u16 5 ("Value (Signaling)")) -> ()  [unwired: 2 in, 2 out]
                n2366 = property on="Background substract" class="Enum (strict)"("Visible"=w2852) -> ()  [unwired: 2 in, 2 out]
                n2367 = property on="CCD ROI" class="Enum (strict)"("Visible"=w2852) -> ()  [unwired: 2 in, 2 out]
                n2368 = property on="Accumulations" class="DigNum (strict)"("Visible"=w2852) -> ()  [unwired: 2 in, 2 out]
                n2369 = property on="CCD 2D Image Main" class="IntGraph (strict)"("Visible"=w2852) -> ()  [unwired: 2 in, 2 out]
                n2370 = property on="CCD 2D Image XY Map" class="IntGraph (strict)"("Visible"=w2852) -> ()  [unwired: 2 in, 2 out]
                n2371 = property on="Exposure Time (ms)" class="DigNum (strict)"("Visible"=w2852) -> ()  [unwired: 2 in, 2 out]
              }
              frame "APD 2" {
                w2854 = FALSE
                w2855 = TRUE
                n2372 = property on="CCD 1D Spectrum XY Map" class="WFGraph (strict)"("Visible"=w2855) -> ()  [unwired: 2 in, 2 out]
                n2373 = property on="CCD 1D Spectrum Main" class="XYGraph (strict)"("Visible"=w2855) -> ()  [unwired: 2 in, 2 out]
                n2374 = property on="Background substract" class="Enum (strict)"("Visible"=w2854) -> ()  [unwired: 2 in, 2 out]
                n2375 = property on="CCD ROI" class="Enum (strict)"("Visible"=w2854) -> ()  [unwired: 2 in, 2 out]
                n2376 = property on="Accumulations" class="DigNum (strict)"("Visible"=w2854) -> ()  [unwired: 2 in, 2 out]
                n2377 = property on="CCD 2D Image Main" class="IntGraph (strict)"("Visible"=w2854) -> ()  [unwired: 2 in, 2 out]
                n2378 = property on="CCD 2D Image XY Map" class="IntGraph (strict)"("Visible"=w2854) -> ()  [unwired: 2 in, 2 out]
                n2379 = property on="Exposure Time (ms)" class="DigNum (strict)"("Visible"=w2854) -> ()  [unwired: 2 in, 2 out]
              }
              frame "APD 1+2" {
                w2857 = FALSE
                w2858 = TRUE
                n2380 = property on="CCD 1D Spectrum XY Map" class="WFGraph (strict)"("Visible"=w2858) -> ()  [unwired: 2 in, 2 out]
                n2381 = property on="CCD 1D Spectrum Main" class="XYGraph (strict)"("Visible"=w2858) -> ()  [unwired: 2 in, 2 out]
                n2382 = property on="Background substract" class="Enum (strict)"("Visible"=w2857) -> ()  [unwired: 2 in, 2 out]
                n2383 = property on="Accumulations" class="DigNum (strict)"("Visible"=w2857) -> ()  [unwired: 2 in, 2 out]
                n2384 = property on="Exit mirror" class="Ring (strict)"("Val(Sgnl)"=u16 5 ("Value (Signaling)")) -> ()  [unwired: 2 in, 2 out]
                n2385 = property on="CCD ROI" class="Enum (strict)"("Visible"=w2857) -> ()  [unwired: 2 in, 2 out]
                n2386 = property on="CCD 2D Image Main" class="IntGraph (strict)"("Visible"=w2857) -> ()  [unwired: 2 in, 2 out]
                n2387 = property on="CCD 2D Image XY Map" class="IntGraph (strict)"("Visible"=w2857) -> ()  [unwired: 2 in, 2 out]
                n2388 = property on="Exposure Time (ms)" class="DigNum (strict)"("Visible"=w2857) -> ()  [unwired: 2 in, 2 out]
              }
            }
            n2389 = local write "Background taken?"(FALSE ("Background taken?")) -> ()
          }
          event "Acq Time (ms)": Value Change {
            n2390 = event-data() -> ("NewVal"=w2860:dbl)  [unwired: 1 in, 5 out]
            n2391 = local read "Acq Mode"() -> (w2861:T3)
            n2392 = case shown="\"Spectrum\", Default" w2861 {
              tunnel: w2860 -> [w2862 w2863]
              frame "Image" {
                n2393 = property on="Exposure Time (ms)" class="DigNum (strict)"("Val(Sgnl)"=w2862) -> ()  [unwired: 2 in, 2 out]
              }
              frame "Spectrum", Default {
                n2394 = property on="Exposure Time (ms)" class="DigNum (strict)"("Val(Sgnl)"=w2863) -> ()  [unwired: 2 in, 2 out]
              }
            }
            n2395 = local write "Background taken?"(FALSE ("Background taken?")) -> ()
          }
          event "Att Amp", "Att Freq", "Att DCLvl", "ANC Axis": Value Change {
            n2396 = event-data() -> ("CtlRef"=w2871:refnum<vi>)  [unwired: 1 in, 5 out]
            n2397 = local read "Att DeviceHandle"() -> (w2868:u64)
            n2398 = property class="Num"(reference=w2871) -> ("Label.Text"=w2870:string)  [unwired: 1 in, 2 out]
            n2399 = local read "ANC Axis"() -> (w2864:u8)
            n2400 = local read "Att Error"() -> (w2869:errorcluster)
            n2401 = local read "ourDLL"() -> (w2865:path)
            n2402 = case shown="\"ANC Axis\", Default" w2870 {
              tunnel: w2869 -> [w2877 w2883 w2891 w2900]
              tunnel: w2868 -> [w2878 w2884 w2892 w2899]
              tunnel: [w2876 w2882 w2890 w2897] -> w2867
              tunnel: [w2875 w2881 w2889 w2898] -> w2866
              tunnel: w2865 -> [w2874 w2885 w2887 w2896]
              tunnel: w2864 -> [w2872 w2879 w2886 w2893]
              frame "Att Freq" {
                n2403 = local read "Att Freq"() -> (w2873:dbl)
                n2404 = call-poly "ANC350v4_Frequency.vi"("deviceHandle"=w2878, "Path to *.DLL"=w2874, "axis"=w2872, "Frequency [Hz] in"=w2873, "error in"=w2877) -> ("deviceHandle"=w2875:u64, "error ANC350v4_frequency"=w2876:errorcluster)  [unwired: 8 in, 1 out]
              }
              frame "Att Amp" {
                n2405 = local read "Att Amp"() -> (w2880:dbl)
                n2406 = call-poly "ANC350v4_Amplitude.vi"("deviceHandle"=w2884, "Path to *.DLL"=w2885, "axis"=w2879, "amplitude in"=w2880, "error in"=w2883) -> ("deviceHandle"=w2881:u64, "error ANC350v4_Amplitude"=w2882:errorcluster)  [unwired: 8 in, 1 out]
              }
              frame "Att DCLvl" {
                n2407 = local read "Att DCLvl"() -> (w2888:dbl)
                n2408 = call "ANC350v4_SetDCVoltage.vi"("deviceHandle"=w2892, "Path to *.DLL"=w2887, "axis"=w2886, "DC voltage"=w2888, "error in"=w2891) -> ("deviceHandle"=w2889:u64, "error ANC350v4_setDCVoltage"=w2890:errorcluster)  [unwired: 8 in, 1 out]
              }
              frame "ANC Axis", Default {
                n2409 = call "ANC350v4_GetDcVoltage.vi"("deviceHandle"=w2899, "Path to *.DLL"=w2896, "axis"=w2893, "error in"=w2900) -> ("deviceHandle"=w2902:u64, "voltage"=w2901:dbl, "error ANC350v4_getDcVoltage"=w2905:errorcluster)  [unwired: 8 in, 1 out]
                n2410 = local write "Att DCLvl"(w2901) -> ()
                n2411 = call-poly "ANC350v4_Frequency.vi"("deviceHandle"=w2902, "Path to *.DLL"=w2896, "axis"=w2893, "error in"=w2905) -> ("deviceHandle"=w2903:u64, "Frequency [Hz] out"=w2895:dbl, "error ANC350v4_frequency"=w2904:errorcluster)  [unwired: 8 in, 1 out]
                n2412 = local write "Att Freq"(w2895) -> ()
                n2413 = call-poly "ANC350v4_Amplitude.vi"("deviceHandle"=w2903, "Path to *.DLL"=w2896, "axis"=w2893, "error in"=w2904) -> ("deviceHandle"=w2898:u64, "amplitude out"=w2894:dbl, "error ANC350v4_Amplitude"=w2897:errorcluster)  [unwired: 8 in, 1 out]
                n2414 = local write "Att Amp"(w2894) -> ()
              }
            }
            n2415 = local write "Att DeviceHandle"(w2866) -> ()
            n2416 = local write "Att Error"(w2867) -> ()
          }
          event "Att Pos X", "Att Pos Y", "Att Pos Z": Value Change {
            n2417 = event-data() -> ("CtlRef"=w2908:refnum<vi>, "NewVal"=w2906:dbl)  [unwired: 1 in, 4 out]
            n2418 = local read "Att Mode"() -> (w2907:enum16{"Single Step", "Continuous", "Automatic"})
            n2419 = flat-sequence {
              tunnel: w2908 -> [w2911]
              tunnel: w2907 -> [w2910]
              tunnel: w2906 -> [w2909]
              frame #0 {
                n2420 = case shown="\"Automatic\"" w2910 {
                  tunnel: w2911 -> [_ w2921]
                  tunnel: w2909 -> [_ w2919]
                  frame "Single Step", Default {
                  }
                  frame "Automatic" {
                    n2421 = property class="DigNum (strict)"(reference=w2921) -> ("Label.Text"=w2920:string)  [unwired: 1 in, 2 out]
                    n2422 = local read "Att DeviceHandle"() -> (w2915:u64)
                    n2423 = local read "Att Error"() -> (w2914:errorcluster)
                    n2424 = case shown="\"Att Pos X\", Default" w2920 {
                      tunnel: [w2923 w2925 w2927] -> w2918
                      tunnel: [w2922 w2924 w2926] -> _
                      frame "Att Pos X", Default {
                        w2923 = u8 1 items=["1", "2", "3"] ("axis")
                        n2425 = control-ref of="Att Pos X"() -> (w2922:refnum<vi>)
                      }
                      frame "Att Pos Y" {
                        w2925 = u8 0 items=["1", "2", "3"] ("axis")
                        n2426 = control-ref of="Att Pos Y"() -> (w2924:refnum<vi>)
                      }
                      frame "Att Pos Z" {
                        w2927 = u8 2 items=["1", "2", "3"] ("axis")
                        n2427 = control-ref of="Att Pos Z"() -> (w2926:refnum<vi>)